vi "HFRR ADV v037.vi"() -> ()   [LabVIEW 2025] (continued)
            n2169 = Match Pattern(string=w2585, regular expression="Frequency :- ") -> (after substring=w2606:string)  [unwired: 1 in, 3 out]
            n2170 = String Subset(string=w2602, length (rest)=6 ("length (rest)")) -> (substring=w2604:string)  [unwired: 1 in]
            n2171 = String Subset(string=w2621, length (rest)=9 ("length (rest)")) -> (substring=w2623:string)  [unwired: 1 in]
            n2172 = String Subset(string=w2598, length (rest)=6 ("length (rest)")) -> (substring=w2600:string)  [unwired: 1 in]
            n2173 = String Subset(string=w2616, length (rest)=9 ("length (rest)")) -> (substring=w2618:string)  [unwired: 1 in]
            n2174 = String Subset(string=w2594, length (rest)=6 ("length (rest)")) -> (substring=w2596:string)  [unwired: 1 in]
            n2175 = String Subset(string=w2611, length (rest)=9 ("length (rest)")) -> (substring=w2613:string)  [unwired: 1 in]
            n2176 = String Subset(string=w2590, length (rest)=6 ("length (rest)")) -> (substring=w2592:string)  [unwired: 1 in]
            n2177 = String Subset(string=w2606, length (rest)=9 ("length (rest)")) -> (substring=w2608:string)  [unwired: 1 in]
            n2178 = Fract/Exp String To Number(string=w2604) -> (number=w2584:dbl)  [unwired: 3 in, 1 out]
            n2179 = Fract/Exp String To Number(string=w2623) -> (number=w2624:dbl)  [unwired: 3 in, 1 out]
            n2180 = Fract/Exp String To Number(string=w2600) -> (number=w2583:dbl)  [unwired: 3 in, 1 out]
            n2181 = Fract/Exp String To Number(string=w2618) -> (number=w2619:dbl)  [unwired: 3 in, 1 out]
            n2182 = Fract/Exp String To Number(string=w2596) -> (number=w2582:dbl)  [unwired: 3 in, 1 out]
            n2183 = Fract/Exp String To Number(string=w2613) -> (number=w2614:dbl)  [unwired: 3 in, 1 out]
            n2184 = Fract/Exp String To Number(string=w2592) -> (number=w2581:dbl)  [unwired: 3 in, 1 out]
            n2185 = Fract/Exp String To Number(string=w2608) -> (number=w2609:dbl)  [unwired: 3 in, 1 out]
            n2186 = local write "sample1"(w2584) -> ()
            n2187 = local write "freq1"(w2624) -> ()
            n2188 = local write "sample2"(w2583) -> ()
            n2189 = local write "freq2"(w2619) -> ()
            n2190 = local write "sample3"(w2582) -> ()
            n2191 = local write "freq3"(w2614) -> ()
            n2192 = local write "sample4"(w2581) -> ()
            n2193 = local write "freq 4"(w2609) -> ()
          }
        }
      }
    }
    n2194 = case shown="True" w2182 {
      selector: w2182 -> [_ w2201]
      frame False {
      }
      frame True {
        n2195 = Not(x=w2201) -> (.not. x?=w2197:bool)
        n2196 = local write "service 3"(w2197) -> ()
        n2197 = local write "OPEN 6"(w2197) -> ()
        n2198 = call <vilib>:"System Exec.vi"("wait until completion? (T)"=TRUE, "command line"="C:\\LAB-IQ\\Scar View.exe") -> ("error out"=→"error out 5":errorcluster)  [unwired: 6 in, 3 out]
      }
    }
    n2199 = case shown="\"Acquire\", Default" w2191 {
      frame "Acquire", Default {
        # "Elapsed time\ncof\nstroke\nAir temp\nTemp\nHumidity"
        n2200 = disable-structure shown="Disabled" {
          frame Disabled {
            n2201 = local read "Flag"() -> (w2900:dbl)
            n2202 = local read "RUN"() -> (w2897:bool)
            n2203 = Not(x=w2897) -> (.not. x?=w2896:bool)
            n2204 = Equal?(x=w2900, y=10.0) -> (x = y?=w2898:bool)
            n2205 = And(x=w2898, y=w2896) -> (x .and. y?=w2895:bool)
            n2206 = case shown="True" w2895 {
              frame False {
              }
              frame True {
                w2901 = FALSE ("Heater Button")
                n2207 = local write "Humidity"(w2901) -> ()
                n2208 = local write "Heater Button"(w2901) -> ()
              }
            }
          }
          frame Enabled {
          }
        }
        n2209 = disable-structure shown="Disabled" {
          frame Disabled {
            n2210 = case shown="True" {
              selector: _ -> [_ _]
              frame False {
              }
              frame True {
                w2946 = TRUE ("Heater")
                n2211 = local write "Humidity"(w2946) -> ()
                n2212 = local write "Heater Button"(w2946) -> ()
                n2213 = local read "TEST STANDARD"() -> (w2949:T3)
                n2214 = local read "TEST STANDARD"() -> (w2944:T3)
                n2215 = Equal?(x=w2949, y=enum16{"ASTM D6079", "ISO 12156", "Custom"}."ISO 12156" ("Test Standard")) -> (x = y?=w2947:bool)
                n2216 = Equal?(x=w2944, y=enum16{"ASTM D6079", "ISO 12156", "Custom"}."ASTM D6079" ("Test Standard")) -> (x = y?=w2943:bool)
                n2217 = case shown="True" w2947 {
                  frame False {
                  }
                  frame True {
                    n2218 = local write "airtempflg"(FALSE ("airtempflg")) -> ()
                    n2219 = local write item#-1(TRUE ("Heater")) -> ()
                  }
                }
                n2220 = case shown="True" w2943 {
                  frame False {
                  }
                  frame True {
                    n2221 = local write "airtempflg"(TRUE ("airtempflg")) -> ()
                    n2222 = local write item#-1(FALSE ("Heater")) -> ()
                  }
                }
              }
            }
          }
          frame Enabled {
          }
        }
        n2223 = stacked-sequence {
          frame #0 {
            n2224 = case shown="True" "RST FF" {
              frame False {
              }
              frame True {
                w2963 = 0.0 ("X Scale.Range:Maximum")
                n2225 = property on="Frictional Force ( N )" class="WFChart (strict)"("XScale.Maximum"=600.0 ("X Scale.Range:Maximum"), "XScale.Minimum"=w2963, "YScale.Maximum"=10.0 ("Y Scale.Range:Maximum"), "YScale.Minimum"=w2963) -> ()  [unwired: 2 in, 2 out]
              }
            }
          }
          frame #1 {
            n2226 = case shown="True" "RST TEMP" {
              frame False {
              }
              frame True {
                n2227 = property on="Temperature ( Deg C )" class="WFChart (strict)"("XScale.Minimum"=0.0 ("X Scale.Range:Minimum"), "XScale.Maximum"=600.0 ("X Scale.Range:Maximum"), "YScale.Minimum"=0.0 ("Y Scale.Range:Minimum"), "YScale.Maximum"=100.0 ("Y Scale.Range:Maximum")) -> ()  [unwired: 2 in, 2 out]
              }
            }
          }
          frame #2 {
            n2228 = case shown="True" "RSTCOF" {
              frame False {
              }
              frame True {
                n2229 = property on="Coefficient of Friction" class="WFChart (strict)"("XScale.Minimum"=0.0 ("X Scale.Range:Minimum"), "XScale.Maximum"=600.0 ("X Scale.Range:Maximum"), "YScale.Maximum"=1.0 ("X Scale.Range:Minimum"), "YScale.Minimum"=0.0 ("X Scale.Range:Minimum")) -> ()  [unwired: 2 in, 2 out]
              }
            }
          }
          frame #3 {
            n2230 = case shown="True" "RSTCOF 2" {
              frame False {
              }
              frame True {
                (unwired) 100.0 ("Y Scale.Range:Maximum")
                (unwired) 0.0 ("Y Scale.Range:Minimum")
                (unwired) 600.0 ("X Scale.Range:Maximum")
                (unwired) 0.0 ("X Scale.Range:Minimum")
              }
            }
          }
          frame #4 {
            n2231 = case shown="True" "RSTCOF 3" {
              frame False {
              }
              frame True {
                n2232 = property on="Electrical Contact Resistance ( % )" class="WFChart (strict)"("XScale.Minimum"=0.0 ("X Scale.Range:Minimum"), "XScale.Maximum"=600.0 ("X Scale.Range:Maximum"), "YScale.Minimum"=0.0 ("Y Scale.Range:Minimum"), "YScale.Maximum"=100.0 ("Y Scale.Range:Maximum")) -> ()  [unwired: 2 in, 2 out]
              }
            }
          }
        }
        n2233 = local read "RUN"() -> (w2890:bool)
        n2234 = case shown="False" w2890 {
          frame False {
          }
          frame True {
          }
        }
        n2235 = local read "RUN"() -> (w2894:bool)
        n2236 = case shown="False" w2894 {
          tunnel: [FALSE ("TEST RUNNING") TRUE ("TEST RUNNING")] -> w2893
          frame False {
            w2982 = 0.0 ("Flag")
            n2237 = local write "Elapsed time"(0.0 ("elapsedtime")) -> ()
            n2238 = local write "Time Remaining"(w2982) -> ()
            n2239 = local write "Flag"(w2982) -> ()
            n2240 = local write "Remaining Time"(w2982) -> ()
          }
          frame True {
            n2241 = local write "Flag"(10.0 ("Flag")) -> ()
          }
        }
        n2242 = local read "AIR TEMP"() -> (w2888:dbl)
        n2243 = Greater Or Equal?(x=w2888, y=15.0) -> (x >= y?=w2889:bool)
        "powstat" <- w2889
        n2244 = case shown="True" "Save & Continue" {
          frame False {
          }
          frame True {
            n2245 = local read "USER ID"() -> (w3286:string)
            n2246 = local read "FILE"() -> (w3294:string)
            n2247 = String Length(string=w3294) -> (length=w3292:i32)
            n2248 = String Length(string=w3286) -> (length=w3289:i32)
            n2249 = Greater?(x=w3292, y=0) -> (0:w3291:bool)
            n2250 = Greater?(x=w3289, y=0) -> (0:w3288:bool)
            n2251 = And(x=w3291, y=w3288) -> (x .and. y?=w3287:bool)
            n2252 = case shown="True" w3287 {
              frame False {
                n2253 = stacked-sequence {
                  frame #0 {
                    n2254 = One Button Dialog(message="Please Enter a File Name and Operator ID to save data !", button name ("OK")="Ok") -> ()  [unwired: 1 out]
                  }
                  frame #1 {
                    n2255 = local write "Save & Continue"(FALSE ("OK Button")) -> ()
                  }
                }
                n2256 = local write "Save & Continue"(FALSE ("OK Button")) -> ()
              }
              frame True {
                n2257 = stacked-sequence {
                  frame #0 {
                    n2258 = local read "FILE"() -> (w3300:string)
                    n2259 = call "file check.vi"("file name in"=w3300) -> ("file name out"=w3299:string)  [unwired: 9 in, 1 out]
                    n2260 = call <vilib>:"Application Directory.vi"() -> ("Application Directory"=w3310:path)
                    n2261 = Build Path(base path=w3310, name or relative path="data") -> (appended path=w3309:path)
                    n2262 = call <vilib>:"Trim Whitespace.vi"("string"=w3299) -> ("trimmed string"=w3307:string)  [unwired: 1 in]
                    n2263 = call <vilib>:"Trim Whitespace.vi"("string"=w3299) -> ("trimmed string"=w3308:string)  [unwired: 1 in]
                    n2264 = List Folder(path=w3309) -> (folder names=w3305:string[])  [unwired: 3 in, 3 out]
                    n2265 = Match Pattern(string=w3307, regular expression="_(") -> (before substring=w3304:string)  [unwired: 1 in, 3 out]
                    n2266 = for {
                      tunnel: w3305 -> [w3319] mode=indexing
                      tunnel: w3304 -> [w3317]
                      shift-right: [w3315] -> w3302
                      shift-left: bool[] [] -> [w3316]
                      n2267 = Match Pattern(string=w3319, regular expression="_(") -> (before substring=w3318:string)  [unwired: 1 in, 3 out]
                      n2268 = Equal?(x=w3318, y=w3317) -> (x = y?=w3314:bool)
                      n2269 = case shown="True" w3314 {
                        tunnel: w3314 -> [_ w3322]
                        tunnel: w3316 -> [w3321 w3324]
                        tunnel: [w3321 w3323] -> w3315
                        frame False {
                        }
                        frame True {
                          n2270 = Insert Into Array(array=w3324, new element=w3322) -> (w3323:bool[])  [unwired: 1 in]
                        }
                      }
                    }
                    n2271 = Equal?(x=w3305, y=w3304) -> (x = y?=w3313:bool[])
                    n2272 = Or Array Elements(Boolean array=w3313) -> (logical OR=w3312:bool)
                    n2273 = Array Size(array=w3302) -> (size(s)=w3301:i32)
                    n2274 = case shown="True" w3312 {
                      tunnel: w3308 -> [_ w3332]
                      tunnel: w3301 -> [_ w3325]
                      frame False {
                      }
                      frame True {
                        n2275 = Number To Decimal String(number=w3325) -> (decimal integer string=w3328:string)  [unwired: 1 in]
                        n2276 = Search/Split String(string=w3332, search string/char (-)="_(" ("regular expression")) -> (substring before match=w3330:string)  [unwired: 1 in, 2 out]
                        n2277 = Concatenate Strings(w3330, "_(" ("regular expression"), w3328, ")" ("regular expression")) -> (w3326:string)
                        n2278 = local write "FILE"(w3326) -> ()
                      }
                    }
                  }
                  frame #1 {
                    w3335 = 0.0
                    w3348 = cluster{"y":dbl, dbl, "y":dbl}[] [] ("History Data")
                    w3349 = FALSE ("Heater Button")
                    (unwired) ")!" ("string")
                    (unwired) ")" ("string")
                    w3347 = dbl[] [] ("History Data")
                    w3353 = "\r"
                    # "C:\\WinDucom\\Data\\"
                    # "C:\\LAB-IQ-NXT\\data"
                    n2279 = local write "Humidity ( %RH )"(w3335) -> ()
                    n2280 = local write "Frequency ( Hz )"(w3335) -> ()
                    n2281 = local write "Stroke 3"(w3335) -> ()
                    n2282 = local write "speedop"(0.0 ("PIDclk 2")) -> ()
                    n2283 = local write "Set Temp 2"(65.0 ("Set Temp 2")) -> ()
                    n2284 = local write "AIR TEMP"(w3335) -> ()
                    n2285 = local write "clk"(0.0 ("clk")) -> ()
                    n2286 = local write "Stroke 4"(w3335) -> ()
                    n2287 = local write "COF 2"(w3335) -> ()
                    n2288 = local write "TEMP"(w3335) -> ()
                    n2289 = local write "ecr 3"(w3335) -> ()
                    n2290 = local write "FF 3"(w3335) -> ()
                    n2291 = local write "FF 2"(w3335) -> ()
                    n2292 = property on="Coefficient of Friction" class="WFChart (strict)"("History Data"=w3347) -> ()  [unwired: 2 in, 2 out]
                    n2293 = property on="Coefficient of Friction" class="WFChart (strict)"("History Data"=w3347) -> ()  [unwired: 2 in, 2 out]
                    n2294 = property on="Frictional Force ( N )" class="WFChart (strict)"("History Data"=w3347) -> ()  [unwired: 2 in, 2 out]
                    n2295 = property on="Electrical Contact Resistance ( % )" class="WFChart (strict)"("History Data"=w3347) -> ()  [unwired: 2 in, 2 out]
                    n2296 = property on="Electrical Contact Resistance ( % )" class="WFChart (strict)"("History Data"=w3347) -> ()  [unwired: 2 in, 2 out]
                    n2297 = property on="Temperature ( Deg C )" class="WFChart (strict)"("History Data"=w3347) -> ()  [unwired: 2 in, 2 out]
                    n2298 = property on="Frictional Force ( N )" class="WFChart (strict)"("History Data"=w3347) -> ()  [unwired: 2 in, 2 out]
                    n2299 = property on="Coefficient of Friction" class="WFChart (strict)"("History Data"=w3347) -> ()  [unwired: 2 in, 2 out]
                    n2300 = property on="Frictional Force ( N )" class="WFChart (strict)"("History Data"=w3347) -> ()  [unwired: 2 in, 2 out]
                    n2301 = property on="Electrical Contact Resistance ( % )" class="WFChart (strict)"("History Data"=w3347) -> ()  [unwired: 2 in, 2 out]
                    n2302 = property on="Temperature ( Deg C )" class="WFChart (strict)"("History Data"=w3347) -> ()  [unwired: 2 in, 2 out]
                    n2303 = property on="Stroke ( mm )" class="WFChart (strict)"("History Data"=w3348) -> ()  [unwired: 2 in, 2 out]
                    n2304 = property on="Stroke ( mm )" class="WFChart (strict)"("History Data"=w3348) -> ()  [unwired: 2 in, 2 out]
                    n2305 = local write "Humidity"(w3349) -> ()
                    n2306 = local write "Heater Button"(w3349) -> ()
                    n2307 = local read "FILE"() -> (w3343:string)
                    n2308 = disable-structure shown="Enabled" {
                      disable-tunnel: [w3387 _] -> w3334
                      frame Enabled {
                        n2309 = local read "NORMAL LOAD"() -> (w3387:dbl)
                      }
                      frame Disabled {
                      }
                    }
                    n2310 = call "file check.vi"("file name in"=w3343) -> ("error out"=w3346:errorcluster, "file name out"=w3340:string)  [unwired: 9 in]
                    n2311 = call "FILE PATH CREATION.vi"("error in"=w3346, "FILE NAME :"=w3340) -> ("FILE OUT"=w3339:path)  [unwired: 8 in, 1 out]
                    n2312 = Concatenate Strings(w3340, ".dgf" ("Substring")) -> (w3345:string)
                    n2313 = Concatenate Strings(w3340, ".duf" ("Substring")) -> (w3341:string)
                    n2314 = Multiply(x=w3334, y=1.0) -> (x*y=w3366:dbl)
                    n2315 = Build Path(base path=w3339, name or relative path=w3345) -> (appended path=w3338:path)
                    n2316 = Build Path(base path=w3339, name or relative path=w3341) -> (appended path=w3337:path)
                    n2317 = Number To Fractional String(number=w3366, width (-)=i16 5, precision (6)=i16 2) -> (F-format string=w3374:string)  [unwired: 1 in]
                    n2318 = local read "tested by"() -> (w3333:string)
                    n2319 = local read "Fuel Discription :"() -> (w3362:string)
                    n2320 = local read "Batch Ref Num :"() -> (w3351:string)
                    n2321 = Get Date/Time String(date format (0)=enum16{"short", "long", "abbreviated"}."short") -> (date string=w3385:string, time string=w3382:string)  [unwired: 2 in]
                    n2322 = local read "Remarks :"() -> (w3361:string)
                    n2323 = Concatenate Strings("Load :- " ("Substring"), w3374, " grams ," ("Substring")) -> (w3373:string)
                    n2324 = local read "String 41"() -> (w3354:string)
                    n2325 = Concatenate Strings(w3362) -> (w3363:string)
                    n2326 = Concatenate Strings(w3351) -> (w3350:string)
                    n2327 = Concatenate Strings(w3333) -> (w3357:string)
                    n2328 = Concatenate Strings("(" ("Substring"), w3385, ")" ("Substring"), w3382) -> (w3356:string)
                    "concatenated string" <- w3356
                    n2329 = Concatenate Strings(w3361, "," ("string")) -> (w3360:string)
                    n2330 = Concatenate Strings("  TIME;      COF;       STROKE;     AIR TEMP;  TEMP;  HUMIDITY;  ECR; PID-OUT; FREQUENCY" ("Substring"), "\r") -> (w3369:string)
                    n2331 = Concatenate Strings(w3354, w3353, "Fuel Discription :-" ("Substring"), w3363, w3353, w3373, w3353, "Batch Ref Num :-" ("Substring"), w3350, w3353, " Remarks :- " ("Substring"), w3360, w3353, " Date :- " ("Substring"), w3356, w3353, "Tested By :-" ("Substring"), w3357) -> (w3367:string)
                    "REMARKS" <- w3367
                    n2332 = call <vilib>:"Write Characters To File.vi"("append to file? (new file:F)"=FALSE, "character string"=w3369, "file path (dialog if empty)"=w3338) -> ()  [unwired: 2 in, 1 out]
                    n2333 = call <vilib>:"Write Characters To File.vi"("append to file? (new file:F)"=FALSE, "character string"=w3367, "file path (dialog if empty)"=w3337) -> ()  [unwired: 2 in, 1 out]
                  }
                  frame #2 {
                    n2334 = local write "Cycles elapsed"(0 ("Cycles elapsed")) -> ()
                    n2335 = local write "cyclecount"(0 ("cyclecount")) -> ()
                    n2336 = local write "Save & Continue"(FALSE ("OK")) -> ()
                    n2337 = local write "autostrtflg"(TRUE ("autostrtflg")) -> ()
                    n2338 = local write "Save"(FALSE ("Save")) -> ()
                    n2339 = Get Date/Time In Seconds() -> (seconds since 1Jan1904=w3392:timestamp)
                    n2340 = To Double Precision Float(number=w3392) -> (double precision float=w3391:dbl)
                    n2341 = local write "acq timer"(w3391) -> ()
                    n2342 = One Button Dialog(message="Please ensure sample is mounted properly and machine is ready in all aspects for testing !", button name ("OK")="Ok") -> ()  [unwired: 1 out]
                  }
                  frame #3 {
                    n2343 = stacked-sequence {
                      frame #0 {
                        n2344 = local write "Main Dashboard Buttons"(T1."Dashboard" ("Main Dashboard Buttons")) -> ()
                        n2345 = local write "Main Tab"(T2."Acquire" ("Main Tab")) -> ()
                      }
                      frame #1 {
                        n2346 = local write "EVENT LOG"("" ("EVENT LOG")) -> ()
                      }
                      frame #2 {
                        n2347 = Wait (ms)(milliseconds to wait=u32 50) -> ()  [unwired: 1 out]
                      }
                      frame #3 {
                        n2348 = disable-structure shown="Disabled" {
                          frame Disabled {
                            n2349 = local read "EVENT LOG"() -> (w3404:string)
                            n2350 = call "Event Log.vi"("Content"="Test Details", "EVENT LOG"=w3404) -> ("EVENT LOG"=w3403:string)  [unwired: 8 in, 1 out]
                            n2351 = local write "EVENT LOG"(w3403) -> ()
                          }
                          frame Enabled {
                          }
                        }
                      }
                      frame #4 {
                        n2352 = Wait (ms)(milliseconds to wait=u32 50) -> ()  [unwired: 1 out]
                      }
                      frame #5 {
                        n2353 = local read "FILE"() -> (w3406:string)
                        n2354 = Concatenate Strings("File Name :" ("Content"), w3406) -> (w3407:string)
                        n2355 = local read "EVENT LOG"() -> (w3410:string)
                        n2356 = call "Event Log.vi"("Content"=w3407, "EVENT LOG"=w3410) -> ("EVENT LOG"=w3409:string)  [unwired: 8 in, 1 out]
                        n2357 = local write "EVENT LOG"(w3409) -> ()
                      }
                      frame #6 {
                        n2358 = Wait (ms)(milliseconds to wait=u32 50) -> ()  [unwired: 1 out]
                      }
                      frame #7 {
                        n2359 = local read "Batch Ref Num :"() -> (w3412:string)
                        n2360 = Concatenate Strings("Batch Ref No :" ("Content"), w3412) -> (w3413:string)
                        n2361 = local read "EVENT LOG"() -> (w3416:string)
                        n2362 = call "Event Log.vi"("Content"=w3413, "EVENT LOG"=w3416) -> ("EVENT LOG"=w3415:string)  [unwired: 8 in, 1 out]
                        n2363 = local write "EVENT LOG"(w3415) -> ()
                      }
                      frame #8 {
                        n2364 = Wait (ms)(milliseconds to wait=u32 50) -> ()  [unwired: 1 out]
                      }
                      frame #9 {
                        n2365 = local read "tested by"() -> (w3418:string)
                        n2366 = Concatenate Strings("Tested By :" ("Content"), w3418) -> (w3419:string)
                        n2367 = local read "EVENT LOG"() -> (w3422:string)
                        n2368 = call "Event Log.vi"("Content"=w3419, "EVENT LOG"=w3422) -> ("EVENT LOG"=w3421:string)  [unwired: 8 in, 1 out]
                        n2369 = local write "EVENT LOG"(w3421) -> ()
                      }
                      frame #10 {
                        n2370 = Wait (ms)(milliseconds to wait=u32 50) -> ()  [unwired: 1 out]
                      }
                      frame #11 {
                        n2371 = local read "TEST STANDARD"() -> (w3425:T3)
                        n2372 = case shown="\"ASTM D6079\", Default" w3425 {
                          tunnel: ["ASTM D6079" "ISO 12156" "CEC F-096-A-06" "Custom"] -> w3424
                          frame "ASTM D6079", Default {
                          }
                          frame "ISO 12156" {
                          }
                          frame "CEC F-096-A-06" {
                          }
                          frame "Custom" {
                          }
                        }
                        n2373 = Concatenate Strings("Test Standard :" ("Content"), w3424) -> (w3426:string)
                        n2374 = local read "EVENT LOG"() -> (w3429:string)
                        n2375 = call "Event Log.vi"("Content"=w3426, "EVENT LOG"=w3429) -> ("EVENT LOG"=w3428:string)  [unwired: 8 in, 1 out]
                        n2376 = local write "EVENT LOG"(w3428) -> ()
                      }
                      frame #12 {
                        n2377 = Wait (ms)(milliseconds to wait=u32 50) -> ()  [unwired: 1 out]
                      }
                      frame #13 {
                        n2378 = local read "Fuel Discription :"() -> (w3435:string)
                        n2379 = Concatenate Strings("Fuel Description :" ("Content"), w3435) -> (w3436:string)
                        n2380 = local read "EVENT LOG"() -> (w3439:string)
                        n2381 = call "Event Log.vi"("Content"=w3436, "EVENT LOG"=w3439) -> ("EVENT LOG"=w3438:string)  [unwired: 8 in, 1 out]
                        n2382 = local write "EVENT LOG"(w3438) -> ()
                      }
                      frame #14 {
                        n2383 = Wait (ms)(milliseconds to wait=u32 50) -> ()  [unwired: 1 out]
                      }
                      frame #15 {
                        n2384 = local read "Remarks :"() -> (w3441:string)
                        n2385 = Concatenate Strings("Remarks :" ("Content"), w3441) -> (w3442:string)
                        n2386 = local read "EVENT LOG"() -> (w3445:string)
                        n2387 = call "Event Log.vi"("Content"=w3442, "EVENT LOG"=w3445) -> ("EVENT LOG"=w3444:string)  [unwired: 8 in, 1 out]
                        n2388 = local write "EVENT LOG"(w3444) -> ()
                      }
                      frame #16 {
                        n2389 = Wait (ms)(milliseconds to wait=u32 50) -> ()  [unwired: 1 out]
                      }
                      frame #17 {
                        n2390 = local read "USER ID"() -> (w3447:string)
                        n2391 = Concatenate Strings("Operator ID :" ("Content"), w3447) -> (w3449:string)
                        n2392 = local read "EVENT LOG"() -> (w3451:string)
                        n2393 = call "Event Log.vi"("Content"=w3449, "EVENT LOG"=w3451) -> ("EVENT LOG"=w3450:string)  [unwired: 8 in, 1 out]
                        n2394 = local write "EVENT LOG"(w3450) -> ()
                      }
                      frame #18 {
                        n2395 = Wait (ms)(milliseconds to wait=u32 50) -> ()  [unwired: 1 out]
                      }
                      frame #19 {
                        n2396 = disable-structure shown="Disabled" {
                          frame Disabled {
                            n2397 = local read "EVENT LOG"() -> (w3455:string)
                            n2398 = call "Event Log.vi"("Content"="Test Parameter", "EVENT LOG"=w3455) -> ("EVENT LOG"=w3454:string)  [unwired: 8 in, 1 out]
                            n2399 = local write "EVENT LOG"(w3454) -> ()
                          }
                          frame Enabled {
                          }
                        }
                      }
                      frame #20 {
                        n2400 = Wait (ms)(milliseconds to wait=u32 50) -> ()  [unwired: 1 out]
                      }
                      frame #21 {
                        n2401 = local read "Set Hz"() -> (w3459:dbl)
                        n2402 = Number To Fractional String(number=w3459, precision (6)=i16 2) -> (F-format string=w3458:string)  [unwired: 2 in]
                        n2403 = Concatenate Strings("Set Frequency [Hz] :" ("Content"), w3458) -> (w3461:string)
                        n2404 = local read "EVENT LOG"() -> (w3463:string)
                        n2405 = call "Event Log.vi"("Content"=w3461, "EVENT LOG"=w3463) -> ("EVENT LOG"=w3462:string)  [unwired: 8 in, 1 out]
                        n2406 = local write "EVENT LOG"(w3462) -> ()
                      }
                      frame #22 {
                        n2407 = Wait (ms)(milliseconds to wait=u32 50) -> ()  [unwired: 1 out]
                      }
                      frame #23 {
                        n2408 = local read "NORMAL LOAD"() -> (w3466:dbl)
                        n2409 = Number To Fractional String(number=w3466, precision (6)=i16 2) -> (F-format string=w3467:string)  [unwired: 2 in]
                        n2410 = Concatenate Strings("Applied Load [grams] :" ("Content"), w3467) -> (w3469:string)
                        n2411 = local read "EVENT LOG"() -> (w3471:string)
                        n2412 = call "Event Log.vi"("Content"=w3469, "EVENT LOG"=w3471) -> ("EVENT LOG"=w3470:string)  [unwired: 8 in, 1 out]
                        n2413 = local write "EVENT LOG"(w3470) -> ()
                      }
                      frame #24 {
                        n2414 = Wait (ms)(milliseconds to wait=u32 50) -> ()  [unwired: 1 out]
                      }
                      frame #25 {
                        n2415 = local read "Set Strk"() -> (w3474:dbl)
                        n2416 = Number To Fractional String(number=w3474, precision (6)=i16 2) -> (F-format string=w3475:string)  [unwired: 2 in]
                        n2417 = Concatenate Strings("Set Stroke [mm] :" ("Content"), w3475) -> (w3477:string)
                        n2418 = local read "EVENT LOG"() -> (w3479:string)
                        n2419 = call "Event Log.vi"("Content"=w3477, "EVENT LOG"=w3479) -> ("EVENT LOG"=w3478:string)  [unwired: 8 in, 1 out]
                        n2420 = local write "EVENT LOG"(w3478) -> ()
                      }
                      frame #26 {
                        n2421 = Wait (ms)(milliseconds to wait=u32 50) -> ()  [unwired: 1 out]
                      }
                      frame #27 {
                        n2422 = local read "Set Temp"() -> (w3482:dbl)
                        n2423 = Number To Fractional String(number=w3482, precision (6)=i16 2) -> (F-format string=w3483:string)  [unwired: 2 in]
                        n2424 = Concatenate Strings("Set Temperature [deg C] :" ("Content"), w3483) -> (w3485:string)
                        n2425 = local read "EVENT LOG"() -> (w3487:string)
                        n2426 = call "Event Log.vi"("Content"=w3485, "EVENT LOG"=w3487) -> ("EVENT LOG"=w3486:string)  [unwired: 8 in, 1 out]
                        n2427 = local write "EVENT LOG"(w3486) -> ()
                      }
                      frame #28 {
                        n2428 = Wait (ms)(milliseconds to wait=u32 50) -> ()  [unwired: 1 out]
                      }
                      frame #29 {
                        n2429 = local read "Set Rh"() -> (w3490:dbl)
                        n2430 = Number To Fractional String(number=w3490, precision (6)=i16 2) -> (F-format string=w3491:string)  [unwired: 2 in]
                        n2431 = Concatenate Strings("Set Humidity [%RH] :" ("Content"), w3491) -> (w3493:string)
                        n2432 = local read "EVENT LOG"() -> (w3495:string)
                        n2433 = call "Event Log.vi"("Content"=w3493, "EVENT LOG"=w3495) -> ("EVENT LOG"=w3494:string)  [unwired: 8 in, 1 out]
                        n2434 = local write "EVENT LOG"(w3494) -> ()
                      }
                      frame #30 {
                        n2435 = Wait (ms)(milliseconds to wait=u32 50) -> ()  [unwired: 1 out]
                      }
                      frame #31 {
                        n2436 = local read "test time"() -> (w3498:dbl)
                        n2437 = Number To Fractional String(number=w3498, precision (6)=i16 1) -> (F-format string=w3499:string)  [unwired: 2 in]
                        n2438 = Concatenate Strings("Test Duration [mins] :" ("Content"), w3499) -> (w3501:string)
                        n2439 = local read "EVENT LOG"() -> (w3503:string)
                        n2440 = call "Event Log.vi"("Content"=w3501, "EVENT LOG"=w3503) -> ("EVENT LOG"=w3502:string)  [unwired: 8 in, 1 out]
                        n2441 = local write "EVENT LOG"(w3502) -> ()
                      }
                      frame #32 {
                        w3504 = dbl[] [] ("History Data")
                        w3505 = cluster{"y":dbl, dbl, "y":dbl}[] [] ("History Data")
                        w3506 = FALSE ("Visible")
                        n2442 = property on="Stroke ( mm )" class="WFChart (strict)"("History Data"=w3505) -> ()  [unwired: 2 in, 2 out]
                        n2443 = property on="Temperature ( Deg C )" class="WFChart (strict)"("History Data"=w3504) -> ()  [unwired: 2 in, 2 out]
                        n2444 = property on="Electrical Contact Resistance ( % )" class="WFChart (strict)"("History Data"=w3504) -> ()  [unwired: 2 in, 2 out]
                        n2445 = property on="Coefficient of Friction" class="WFChart (strict)"("History Data"=w3504) -> ()  [unwired: 2 in, 2 out]
                        n2446 = property on="Frictional Force ( N )" class="WFChart (strict)"("History Data"=w3504) -> ()  [unwired: 2 in, 2 out]
                        n2447 = property on="Coefficient of Friction" class="WFChart (strict)"("History Data"=w3504) -> ()  [unwired: 2 in, 2 out]
                        n2448 = property on="Frictional Force ( N )" class="WFChart (strict)"("History Data"=w3504) -> ()  [unwired: 2 in, 2 out]
                        n2449 = property on="Electrical Contact Resistance ( % )" class="WFChart (strict)"("History Data"=w3504) -> ()  [unwired: 2 in, 2 out]
                        n2450 = property on="Stroke ( mm )" class="WFChart (strict)"("History Data"=w3505) -> ()  [unwired: 2 in, 2 out]
                        n2451 = property on="Temperature ( Deg C )" class="WFChart (strict)"("History Data"=w3504) -> ()  [unwired: 2 in, 2 out]
                        n2452 = property on="Service Password Log" class="Str"("Visible"=w3506) -> ()  [unwired: 2 in, 2 out]
                        n2453 = property on="Password 3" class="Clust (strict)"("Visible"=w3506) -> ()  [unwired: 2 in, 2 out]
                      }
                    }
                    "TEST FILE NAM,E SAVED" <- TRUE ("TEST FILE NAM,E SAVED")
                  }
                }
              }
            }
          }
        }
        n2454 = local write "Test \nStatus"(w2893) -> ()
        n2455 = local write "Save"(w2893) -> ()
        n2456 = local read "Main Tab"() -> (w2887:T2)
        n2457 = case shown="True" w2890 {
          frame False {
            n2458 = local read "Rt 3"() -> (w2954:bool)
            n2459 = case shown="True" w2954 {
              frame False {
              }
              frame True {
                n2460 = local write "Rt 3"(FALSE ("Rt 3")) -> ()
              }
            }
            "Rt" <- TRUE ("Rt")
            "Rt 2" <- FALSE ("Rt")
          }
          frame True {
            n2461 = local read "Rt"() -> (w2960:bool)
            n2462 = local write "Rt 2"(TRUE ("Rt 2")) -> ()
            n2463 = case shown="True" w2960 {
              frame False {
              }
              frame True {
                n2464 = local write "Rt"(FALSE ("Rt")) -> ()
              }
            }
            "Rt 3" <- TRUE ("Rt 3")
          }
        }
        n2465 = case shown="\"Acquire\"" w2887 {
          tunnel: w2889 -> [_ w2989]
          frame Default {
            w2988 = 0.0 ("output")
            n2466 = local write "PID-out"(w2988) -> ()
            n2467 = local write "Frequency ( Hz )"(w2988) -> ()
            n2468 = local write "STROKE Initialize"(TRUE ("STROKE Initialize")) -> ()
          }
          frame "Acquire" {
            n2469 = stacked-sequence {
              frame #0 {
                n2470 = local read "Auto Start Test"() -> (w2991:bool)
                n2471 = case shown="True" w2991 {
                  tunnel: "RUN" -> [w3012 w3015]
                  tunnel: [w3012 w3014] -> w2992
                  frame False {
                  }
                  frame True {
                    n2472 = local read "Auto Start Temp"() -> (w3013:bool)
                    n2473 = Or(x=w3015, y=w3013) -> (x .or. y?=w3014:bool)
                  }
                }
                n2474 = local read "clk"() -> (w3011:dbl)
                n2475 = local read "Save"() -> (w3007:bool)
                n2476 = Equal?(x=w3011, y=0.0) -> (x = y?=w3008:bool)
                n2477 = And(x=w3008, y=w3007) -> (x .and. y?=w3009:bool)
                n2478 = Not(x="Engage") -> (.not. x?=w2998:bool)
                n2479 = case shown="False" w2992 {
                  tunnel: [0.0 w3039] -> w2994
                  frame False {
                    (unwired) TRUE ("Visible")
                    n2480 = local read "Auto Start Test"() -> (w3019:bool)
                    n2481 = local write "Start Time"(TRUE ("Start Time")) -> ()
                    n2482 = property on="Stroke 2" class="DigNum (strict)"("Visible"=FALSE) -> ()  [unwired: 2 in, 2 out]
                    n2483 = case shown="False" w3019 {
                      frame False {
                        n2484 = property on="Heater Button" class="Bool (strict)"("DisabledEnum"=T19."Enabled" ("Disabled")) -> ()  [unwired: 2 in, 2 out]
                        n2485 = property on="Humidity" class="Bool (strict)"("DisabledEnum"=T19."Enabled" ("Disabled")) -> ()  [unwired: 2 in, 2 out]
                      }
                      frame True {
                      }
                    }
                    n2486 = case shown="False" "TestCompFlg" {
                      frame False {
                        n2487 = local read "StartFlg"() -> (w3027:bool)
                        n2488 = case shown="True" w3027 {
                          frame False {
                          }
                          frame True {
                            n2489 = stacked-sequence {
                              frame #0 {
                                n2490 = local read "EVENT LOG"() -> (w3031:string)
                                n2491 = call "Event Log.vi"("Content"="Test was interrupted", "EVENT LOG"=w3031) -> ("EVENT LOG"=w3032:string)  [unwired: 8 in, 1 out]
                                n2492 = local write "EVENT LOG"(w3032) -> ()
                                n2493 = property on="RUN" class="Bool (strict)"("Visible"=TRUE) -> ()  [unwired: 2 in, 2 out]
                                n2494 = property on="Auto Start Test" class="Bool (strict)"("Visible"=TRUE) -> ()  [unwired: 2 in, 2 out]
                              }
                              frame #1 {
                                w3035 = FALSE ("StartFlg")
                                n2495 = property on="Heater Button" class="Bool (strict)"("Val(Sgnl)"=FALSE ("Value (Signaling)")) -> ()  [unwired: 2 in, 2 out]
                                n2496 = local write "Heater Button"(w3035) -> ()
                                n2497 = local write "StartFlg"(w3035) -> ()
                                n2498 = local write "Humidity"(w3035) -> ()
                                n2499 = local write "Humidity"(TRUE ("Humidity")) -> ()
                              }
                              frame #2 {
                                n2500 = local write "Due Write"("VC;0" ("Command")) -> ()
                              }
                              frame #3 {
                                n2501 = Wait (ms)(milliseconds to wait=u32 1500) -> ()  [unwired: 1 out]
                              }
                              frame #4 {
                                n2502 = local write "Due Write"("HE;0" ("Command")) -> ()
                              }
                            }
                          }
                        }
                      }
                      frame True {
                      }
                    }
                    n2503 = local write "String 14"("Test will autostart once parameters reach the set value." ("String 14")) -> ()
                  }
                  frame True {
                    (unwired) FALSE ("Visible")
                    n2504 = property on="Stroke 2" class="DigNum (strict)"("Visible"=TRUE) -> ()  [unwired: 2 in, 2 out]
                    n2505 = property on="STOP 2" class="Bool (strict)"("Disabled"=u8 2) -> ()  [unwired: 2 in, 2 out]
                    n2506 = local write "String 14"(" Running....." ("String 14")) -> ()
                    n2507 = property on="Heater Button" class="Bool (strict)"("DisabledEnum"=T19."Disabled and Grayed Out" ("Disabled")) -> ()  [unwired: 2 in, 2 out]
                    n2508 = property on="Humidity" class="Bool (strict)"("DisabledEnum"=T19."Disabled and Grayed Out" ("Disabled")) -> ()  [unwired: 2 in, 2 out]
                    n2509 = case shown="True" "Start Time" {
                      selector: "Start Time" -> [_ w3058]
                      frame False {
                      }
                      frame True {
                        n2510 = Not(x=w3058) -> (.not. x?=w3057:bool)
                        n2511 = local write "Start Time"(w3057) -> ()
                        n2512 = local read "EVENT LOG"() -> (w3059:string)
                        n2513 = call "Event Log.vi"("Content"="Test in progress", "EVENT LOG"=w3059) -> ("EVENT LOG"=w3061:string)  [unwired: 8 in, 1 out]
                        n2514 = local write "EVENT LOG"(w3061) -> ()
                      }
                    }
                    n2515 = disable-structure shown="Enabled" {
                      disable-tunnel: [w3050 w3056] -> w3039
                      frame Disabled {
                        n2516 = local read "Set Hz"() -> (w3053:dbl)
                        n2517 = call <vilib>:"Uniform White Noise Waveform.vi"() -> ("signal out"=w3052:waveform(dbl))  [unwired: 10 in, 1 out]
                        n2518 = Random Number (0-1)() -> (number: 0 to 1=w3049:dbl)
                        n2519 = Add(x=w3053, y=w3052) -> (x+y=w3051:waveform(dbl))
                        n2520 = Multiply(x=ext 0.01 ("y"), y=w3049) -> (x*y=w3047:ext)
                        n2521 = Multiply(x=w3051, y=w3047) -> (x*y=w3050:waveform(ext))
                      }
                      frame Enabled {
                        n2522 = call-poly <vilib>:"Random Number (Range).vi"("lower bound (0)"=49.89, "upper bound (100)"=50.8) -> ("number"=w3056:dbl)  [unwired: 9 in]
                      }
                    }
                    "StartFlg" <- TRUE ("StartFlg")
                  }
                }
                n2523 = case shown="True" w3009 {
                  frame False {
                  }
                  frame True {
                    n2524 = local write "clk"(10.0 ("clk")) -> ()
                    n2525 = Get Date/Time In Seconds() -> (seconds since 1Jan1904=w3064:timestamp)
                    n2526 = To Double Precision Float(number=w3064) -> (double precision float=w3062:dbl)
                    n2527 = local write "acq timer"(w3062) -> ()
                    n2528 = local write "act save time"(w3062) -> ()
                  }
                }
                n2529 = call "Elapsed Time"("Time Target (s)"="Countdown", "Reset"=w2998) -> ("Elapsed Time (s)"=w3003:dbl, "Time has Elapsed"=w3001:bool)  [unwired: 10 in, 6 out]
                "Countdown 2" <- w3003
                n2530 = Subtract(x=w3003, y=2.0) -> (x-y=w3006:dbl)
                n2531 = Less?(x=w3006, y="Countdown") -> (x < y?=w3004:bool)
                n2532 = And(x=w3004, y=w3001) -> (x .and. y?=w3000:bool)
                n2533 = case shown="True" w3000 {
                  frame False {
                  }
                  frame True {
                    (unwired) dbl[] [] ("History Data")
                    n2534 = local write "Engage"(FALSE ("Engage")) -> ()
                    n2535 = local write "RUN"(TRUE ("RUN")) -> ()
                    n2536 = local read "Humidity ( %RH )"() -> (→"Rh Before":dbl)
                  }
                }
                n2537 = local read "Test \nStatus"() -> (w2996:bool)
                n2538 = Select(t=w2994, s=w2996, f=0.0) -> (s? t:f=w2995:dbl)
                n2539 = local write "Frequency ( Hz )"(w2995) -> ()
              }
              frame #1 {
                w3087 = 1000000.0 ("x")
                # "HC;1/0\nST;VALUE"
                # "Elapsed time\ncof\nstroke\nAir temp\nTemp\nHumidity"
                # "acq timer\n\nact save time"
                # "convert to microseconds"
                n2540 = local read "COUNT"() -> (w3070:i32)
                n2541 = local read "Rate"() -> (w3083:dbl)
                n2542 = Divide(x=w3087, y=w3083) -> (x/y=w3088:dbl)
                n2543 = Greater Or Equal?(x=w3070, y=250) -> (x >= y?=w3069:bool)
                n2544 = Get Date/Time In Seconds() -> (seconds since 1Jan1904=w3090:timestamp)
                n2545 = case shown="True" w3069 {
                  frame False {
                    n2546 = local read "COUNT"() -> (w3091:i32)
                    n2547 = Increment(x=w3091) -> (x+1=w3092:i32)
                    n2548 = local write "COUNT"(w3092) -> ()
                  }
                  frame True {
                    n2549 = local write "COUNT"(0 ("COUNT")) -> ()
                  }
                }
                n2550 = local read "Samplingtime 2"() -> (w3068:dbl)
                n2551 = local read "act save time"() -> (w3085:dbl)
                n2552 = Divide(x=w3088, y=w3087) -> (x/y=w3086:dbl)
                n2553 = To Double Precision Float(number=w3090) -> (double precision float=w3079:dbl)
                n2554 = Add(x=w3085, y=w3068) -> (x+y=w3084:dbl)
                n2555 = local read "acq timer"() -> (w3089:dbl)
                n2556 = local read "COUNT"() -> (w3072:i32)
                n2557 = Greater Or Equal?(x=w3079, y=w3084) -> (x >= y?=w3067:bool)
                n2558 = Multiply(x=w3086, y=w3072) -> (x*y=w3078:dbl)
                n2559 = Subtract(x=w3079, y=w3089) -> (x-y=w3081:dbl)
                n2560 = local read "Save"() -> (w3082:bool)
                n2561 = Add(x=w3081, y=w3078) -> (x+y=w3065:dbl)
                "Elapsed time 3" <- w3065
                n2562 = And(x=w3067, y=w3082) -> (x .and. y?=w3080:bool)
                n2563 = Divide(x=w3065, y=60.0) -> (x/y=w3076:dbl)
                n2564 = local read "Test \nStatus"() -> (w3066:bool)
                n2565 = local read "clk"() -> (w3073:dbl)
                n2566 = Equal?(x=w3073, y=10.0) -> (x = y?=w3075:bool)
                n2567 = case shown="True" w3080 {
                  tunnel: w3079 -> [_ w3206]
                  tunnel: [FALSE ("Boolean 2") TRUE ("Boolean 2")] -> _
                  frame False {
                  }
                  frame True {
                    w3160 = ";" ("Substring")
                    # "Pid out/\nFreq response value"
                    n2568 = local write "act save time"(w3206) -> ()
                    n2569 = local read "FILE"() -> (w3154:string)
                    n2570 = call "file check.vi"("file name in"=w3154) -> ("error out"=w3157:errorcluster, "file name out"=w3152:string)  [unwired: 9 in]
                    n2571 = local read "LVDT STROKE"() -> (w3149:dbl)
                    n2572 = local read "Add up Stroke"() -> (w3147:dbl)
                    n2573 = call "FILE PATH CREATION.vi"("error in"=w3157, "FILE NAME :"=w3152) -> ("FILE OUT"=w3155:path)  [unwired: 8 in, 1 out]
                    n2574 = local read "STROKE Initialize"() -> (w3142:bool)
                    n2575 = Concatenate Strings(w3152, ".dgf" ("Substring")) -> (w3156:string)
                    n2576 = Subtract(x=w3149, y=w3147) -> (x-y=w3148:dbl)
                    n2577 = Absolute Value(x=w3148) -> (abs(x)=w3145:dbl)
                    n2578 = local read "FF 2"() -> (→"Frictional Force ( N )" →"Frictional Force ( N )":dbl)
                    n2579 = Build Path(base path=w3155, name or relative path=w3156) -> (appended path=w3151:path)
                    n2580 = flat-sequence {
                      tunnel: w3145 -> [w3211]
                      tunnel: [w3210] -> w3143
                      tunnel: w3142 -> [w3208]
                      tunnel: [w3213] -> w3144
                      tunnel: w3143 -> [w3213]
                      frame #0 {
                        n2581 = call <vilib>:"Mean PtByPt.vi"("x"=w3211, "sample length"="STROKE FILTER", "initialize"=w3208) -> ("mean"=w3210:dbl)  [unwired: 1 in, 1 out]
                      }
                      frame #1 {
                        "STROKE Initialize" <- FALSE ("STROKE Initialize")
                      }
                    }
                    n2582 = local read "COF 2"() -> (w3165:dbl)
                    "Coefficient of Friction" <- w3165
                    "COF 4" <- w3165
                    "Coefficient of Friction" <- w3165
                    n2583 = local read "TEMP"() -> (w3168:dbl)
                    "Temperature ( Deg C )" <- w3168
                    n2584 = local read "Humidity ( %RH )"() -> (w3167:dbl)
                    n2585 = local read "Frequency ( Hz )"() -> (w3174:dbl)
                    n2586 = local read "LVDT STROKE DISPLAY"() -> (w3146:dbl)
                    n2587 = local read "Elapsed time"() -> (w3199:dbl)
                    n2588 = local read "AIR TEMP"() -> (w3172:dbl)
                    n2589 = local read "PID-out"() -> (w3177:dbl)
                    n2590 = local write "Temperature ( Deg C )"(w3168) -> ()
                    n2591 = Number To Fractional String(number=w3146, width (-)=i16 9 ("precision (6)"), precision (6)=i16 6) -> (F-format string=w3192:string)  [unwired: 1 in]
                    n2592 = Number To Fractional String(number=w3172, width (-)=i16 9 ("precision (6)"), precision (6)=i16 3) -> (F-format string=w3191:string)  [unwired: 1 in]
                    n2593 = Number To Fractional String(number=w3168, width (-)=i16 9 ("precision (6)"), precision (6)=i16 3) -> (F-format string=w3188:string)  [unwired: 1 in]
                    n2594 = Number To Fractional String(number=w3167, width (-)=i16 9 ("precision (6)"), precision (6)=i16 3) -> (F-format string=w3185:string)  [unwired: 1 in]
                    n2595 = Number To Fractional String(number=0.0, width (-)=i16 9 ("precision (6)"), precision (6)=i16 3) -> (F-format string=w3182:string)  [unwired: 1 in]
                    n2596 = Number To Fractional String(number=w3177, width (-)=i16 9 ("precision (6)"), precision (6)=i16 3) -> (F-format string=w3178:string)  [unwired: 1 in]
                    n2597 = Number To Fractional String(number=w3174, width (-)=i16 9 ("precision (6)"), precision (6)=i16 3) -> (F-format string=w3173:string)  [unwired: 1 in]
                    n2598 = Number To Fractional String(number=w3165, width (-)=i16 9 ("precision (6)"), precision (6)=i16 6) -> (F-format string=w3200:string)  [unwired: 1 in]
                    n2599 = Number To Fractional String(number=w3199, width (-)=i16 14 ("precision (6)"), precision (6)=i16 3) -> (F-format string=w3201:string)  [unwired: 1 in]
                    n2600 = Bundle("y"=1.02, "LVDT STROKE DISPLAY"=w3146, "y"=0.98) -> (w3166:T31)  [unwired: 1 in]
                    n2601 = Number To Fractional String(number="Ambient Humidity :", width (-)=i16 9 ("precision (6)"), precision (6)=i16 6) -> (F-format string=w3158:string)  [unwired: 1 in]
                    n2602 = local read "RUN"() -> (w3164:bool)
                    n2603 = case shown="True" w3164 {
                      tunnel: w3166 -> [_ w3217]
                      tunnel: w3146 -> [_ w3216]
                      tunnel: w3146 -> [_ w3214]
                      tunnel: w3146 -> [_ w3215]
                      frame False {
                      }
                      frame True {
                        "Stroke ( mm )" <- w3217
                        "Stroke ( mm )" <- w3217
                        "Stroke 4" <- w3216
                        "Stroke 3" <- w3214
                        "Stroke 2" <- w3215
                        "measured_stroke" <- w3214
                      }
                    }
                    n2604 = Concatenate Strings(w3201, w3160, w3200, w3160, w3192, w3160, w3191, w3160, w3188, w3160, w3185, w3160, w3182, w3160, w3178, w3160, w3173, w3160, w3158, "\r") -> (w3198:string)
                    n2605 = call <vilib>:"Write Characters To File.vi"("append to file? (new file:F)"=TRUE, "character string"=w3198, "file path (dialog if empty)"=w3151) -> ()  [unwired: 2 in, 1 out]
                    "refresh flag" <- TRUE ("refresh flag")
                    "LVDT STROKE Actual" <- w3144
                  }
                }
                n2606 = case shown="True" w3066 {
                  tunnel: w3076 -> [_ w3102]
                  tunnel: w3081 -> [_ w3112]
                  tunnel: [0.0 w3108] -> _
                  tunnel: w3075 -> [_ w3107]
                  tunnel: [0.0 w3106] -> _
                  tunnel: w3065 -> [_ w3106]
                  tunnel: w3079 -> [w3095 _]
                  frame False {
                    n2607 = local write "acq timer"(w3095) -> ()
                    n2608 = local write "Test Duration Status"(0.0 ("Test Duration Status")) -> ()
                  }
                  frame True {
                    n2609 = local read "Set Hz"() -> (w3109:dbl)
                    n2610 = local write "Elapsed time"(w3102) -> ()
                    n2611 = local read "test time"() -> (w3101:dbl)
                    n2612 = Multiply(x=w3112, y=w3109) -> (x*y=w3111:dbl)
                    n2613 = case shown="False" w3107 {
                      tunnel: w3111 -> [w3113 _]
                      tunnel: [w3113 1.0] -> w3108
                      frame False {
                        n2614 = local write "Cycles elapsed"(w3113) -> ()
                      }
                      frame True {
                      }
                    }
                    n2615 = Greater?(x=w3102, y=w3101) -> (0:w3110:bool)
                    n2616 = Subtract(x=w3101, y=w3102) -> (x-y=w3100:dbl)
                    n2617 = Multiply(x=w3100, y=60.0) -> (x*y=w3099:dbl)
                    n2618 = local write "Time Remaining"(w3099) -> ()
                    n2619 = local write "Remaining Time"(w3099) -> ()
                    n2620 = case shown="True" w3110 {
                      frame False {
                      }
                      frame True {
                        n2621 = stacked-sequence {
                          frame #0 {
                            w3118 = T19."Enabled" ("Disabled")
                            w3117 = FALSE ("TEST FILE NAM,E SAVED")
                            w3119 = "" ("FILE")
                            w3120 = TRUE ("Visible")
                            n2622 = local write "Humidity"(FALSE ("Humidity")) -> ()
                            n2623 = local write "RUN"(FALSE ("OK Button 2")) -> ()
                            n2624 = local write "Heater Button"(FALSE ("Heater Button")) -> ()
                            n2625 = local write "Auto Start Test"(FALSE ("Auto Start Test")) -> ()
                            n2626 = local write "TestCompFlg"(TRUE ("StpFlg")) -> ()
                            n2627 = local read "Humidity ( %RH )"() -> (→"Rh After":dbl)
                            n2628 = property on="STOP 2" class="Bool (strict)"("Disabled"=u8 0) -> ()  [unwired: 2 in, 2 out]
                            n2629 = local read "EVENT LOG"() -> (w3125:string)
                            n2630 = call "Event Log.vi"("Content"="Test Completed", "EVENT LOG"=w3125) -> ("EVENT LOG"=w3124:string)  [unwired: 8 in, 1 out]
                            n2631 = property on="RUN" class="Bool (strict)"("Visible"=w3120) -> ()  [unwired: 2 in, 2 out]
                            n2632 = property on="Auto Start Test" class="Bool (strict)"("Visible"=w3120) -> ()  [unwired: 2 in, 2 out]